vi "UHR-Fleezers Control (host) - 10.2.vi"() -> ()   [LabVIEW 2009] (continued)
            n295 = Bundle("T1 Y", "T1 X", "T1 Sum", "T2 Y", "T2 X", "T2 Sum", "T1 FB Sum", "T2 FB Sum", "PSD Y", "PSD X", "PSD Y Sum", "PSD X Sum") -> (w2177:T36)  [unwired: 1 out]
            n296 = To Word Integer(number=w2210) -> (16bit integer=w2169:i16[])
            n297 = Cluster To Array(cluster=w2177) -> (array=w2196:string[])
          }
          frame #1 {
            w2277 = 2  # Channel pattern
            # "time average x2 the 3 psd signals (detection laser)"
            # "deinterlace 3 signals from qpds"
            n298 = Decimate 1D Array(w2297) -> (w2296:i16[], w2295:i16[], w2278:i16[], w2294:i16[], w2240:i16[], w2237:i16[], w2234:i16[], w2265:i16[])
            n299 = Decimate 1D Array(w2278) -> (w2263:i16[], w2261:i16[])
            n300 = Decimate 1D Array(w2296) -> (w2293:i16[], w2280:i16[])
            n301 = Decimate 1D Array(w2295) -> (w2292:i16[], w2290:i16[])
            n302 = Decimate 1D Array(w2294) -> (w2291:i16[], w2289:i16[])
            n303 = Decimate 1D Array(w2265) -> (w2264:i16[], w2262:i16[])
            n304 = call "downsample 1D array - I16.vi"("Ave N"=2.0, "Array In"=w2240) -> ("Array Out"=w2238:i16[])  [unwired: 1 in]
            n305 = call "downsample 1D array - I16.vi"("Ave N"=2.0, "Array In"=w2234) -> ("Array Out"=w2232:i16[])  [unwired: 1 in]
            n306 = call "downsample 1D array - I16.vi"("Ave N"=2.0, "Array In"=w2237) -> ("Array Out"=w2235:i16[])  [unwired: 1 in]
            n307 = Interleave 1D Arrays(w2293, w2292, w2291, w2280, w2290, w2289, w2264, w2263, w2262, w2261, w2238, w2235, w2232) -> (w2288:i16[])
            n308 = Divide(x=w2288, y=3276.7) -> (x/y=w2287:dbl[])
            n309 = Decimate 1D Array(w2287) -> (w2286:dbl[], w2285:dbl[], w2284:dbl[], w2283:dbl[], w2282:dbl[], w2281:dbl[], w2253:dbl[], w2251:dbl[], w2250:dbl[], w2248:dbl[], w2247:dbl[], w2246:dbl[], w2243:dbl[])
            n310 = Negate(x=w2243) -> (-x=w2241:dbl[])
            n311 = Divide(x=w2247, y=w2243) -> (x/y=w2245:dbl[])
            n312 = Divide(x=w2246, y=w2241) -> (x/y=w2244:dbl[])
            n313 = Divide(x=w2286, y=w2284) -> (x/y=w2269:dbl[])
            n314 = Divide(x=w2285, y=w2284) -> (x/y=w2268:dbl[])
            n315 = Divide(x=w2283, y=w2281) -> (x/y=w2267:dbl[])
            n316 = Divide(x=w2282, y=w2281) -> (x/y=w2266:dbl[])
            n317 = Divide(x=w2253, y=w2251) -> (x/y=w2252:dbl[])
            n318 = Divide(x=w2250, y=w2248) -> (x/y=w2249:dbl[])
            n319 = Build Array(w2269, w2268, w2284, w2267, w2266, w2281, w2252, w2251, w2249, w2248, w2245, w2244, w2243) -> (w2242:dbl[][])
            n320 = Bundle("T1 Y", "T1 X", "T1 Sum", "T2 Y", "T2 X", "T2 Sum", "T1 FB X", "T1 FB Sum", "T2 FB X", "T2 FB Sum", "PSD Y", "PSD X", "PSD Y Sum") -> (w2270:T37)  [unwired: 1 out]
            n321 = Cluster To Array(cluster=w2270) -> (array=w2279:string[])
          }
          frame #2 {
            w2344 = 4  # Channel pattern
            # "time average x2 the 3 psd signals (detection laser)"
            # "deinterlace 3 signals from qpds"
            n322 = Decimate 1D Array(w2368) -> (w2367:i16[], w2366:i16[], w2345:i16[], w2365:i16[], w2311:i16[], w2357:i16[], w2356:i16[], w2333:i16[])
            n323 = Decimate 1D Array "Feedback Sum"(w2345) -> (w2329:i16[], w2327:i16[])
            n324 = Decimate 1D Array "QPD Y"(w2367) -> (w2364:i16[], w2347:i16[])
            n325 = Decimate 1D Array "QPD X"(w2366) -> (w2363:i16[], w2361:i16[])
            n326 = Decimate 1D Array "Feedback Y"(w2311) -> (w2310:i16[], w2309:i16[])
            n327 = Decimate 1D Array "QPD Sum"(w2365) -> (w2362:i16[], w2360:i16[])
            n328 = Decimate 1D Array "Feedback X"(w2333) -> (w2330:i16[], w2328:i16[])
            n329 = call "downsample 1D array - double.vi"("Ave N"=2.0, "Array In"=w2357) -> ("Array Out"=w2332:dbl[])  [unwired: 1 out]
            n330 = call "downsample 1D array - double.vi"("Ave N"=2.0, "Array In"=w2356) -> ("Array Out"=w2331:dbl[])  [unwired: 1 out]
            n331 = Interleave 1D Arrays(w2364, w2363, w2362, w2347, w2361, w2360, w2310, w2330, w2329, w2309, w2328, w2327, w2332, w2331) -> (w2355:dbl[])
            n332 = Divide(x=w2355, y=3276.7) -> (x/y=w2354:dbl[])
            n333 = Decimate 1D Array(w2354) -> (w2353:dbl[], w2352:dbl[], w2351:dbl[], w2350:dbl[], w2349:dbl[], w2348:dbl[], w2306:dbl[], w2320:dbl[], w2304:dbl[], w2305:dbl[], w2318:dbl[], w2302:dbl[], w2316:dbl[], w2314:dbl[])
            n334 = Negate(x=w2314) -> (-x=w2312:dbl[])
            n335 = Divide(x=w2316, y=w2312) -> (x/y=w2315:dbl[])
            n336 = Divide(x=w2305, y=w2302) -> (x/y=w2301:dbl[])
            n337 = Divide(x=w2306, y=w2304) -> (x/y=w2303:dbl[])
            n338 = Divide(x=w2353, y=w2351) -> (x/y=w2337:dbl[])
            n339 = Divide(x=w2352, y=w2351) -> (x/y=w2336:dbl[])
            n340 = Divide(x=w2350, y=w2348) -> (x/y=w2335:dbl[])
            n341 = Divide(x=w2349, y=w2348) -> (x/y=w2334:dbl[])
            n342 = Divide(x=w2320, y=w2304) -> (x/y=w2319:dbl[])
            n343 = Divide(x=w2318, y=w2302) -> (x/y=w2317:dbl[])
            n344 = Build Array(w2337, w2336, w2351, w2335, w2334, w2348, w2303, w2319, w2304, w2301, w2317, w2302, w2315, w2314) -> (w2313:dbl[][])
            n345 = Bundle("T1 Y", "T1 X", "T1 Sum", "T2 Y", "T2 X", "T2 Sum", "T1 FB Y", "T1 FB X", "T1 FB Sum", "T2 FB Y", "T2 FB X", "T2 FB Sum", "PSD X", "PSD Y Sum") -> (w2300:T38)  [unwired: 1 out]
            n346 = To Word Integer(number=w2355) -> (16bit integer=w2299:i16[])
            n347 = Cluster To Array(cluster=w2300) -> (array=w2346:string[])
          }
        }
      }
    }
    "AI labels" <- w866
    n348 = Decimate 1D Array(w834) -> (w862:u32[], w798:u32[])
    n349 = local read "DMA Update Period (s)"() -> (w876:dbl)
    n350 = local read "BD 1 Frequency 2 (MHz)"() -> (w737:dbl)
    n351 = local read "BD 1 Frequency 1 (MHz)"() -> (w738:dbl)
    n352 = Build Array(w862, w798) -> (w944:u32[][])
    n353 = local read "Data Period (s)"() -> (w847:dbl)
    n354 = Decimate 1D Array(w745) -> (w769:i16[], w768:i16[], w766:i16[], w765:i16[])  [unwired: 9 out]
    n355 = To Double Precision Float(number=w944) -> (double precision float=w945:dbl[][])
    n356 = local read "APD Integration Time (s)"() -> (w811:dbl)
    n357 = Divide(x=w769, y=w768) -> (x/y=w770:dbl[])
    n358 = Divide(x=w766, y=w765) -> (x/y=w767:dbl[])
    n359 = feedback #1(0.0) -> (w783:dbl)
    n360 = Add(x=w876, y=w783) -> (x+y=w984:dbl)
    n361 = local read "AOM X Cal (nm/MHz)"() -> (w735:dbl)
    n362 = To Time Stamp(1:w783) -> (0:w782:timestamp)
    n363 = Split 1D Array(array=w770, index="N El. to Ave.") -> (second subarray=w773:dbl[])  [unwired: 1 out]
    n364 = Split 1D Array(array=w767, index="N El. to Ave.") -> (second subarray=w772:dbl[])  [unwired: 1 out]
    n365 = local read "Trap X AI1 (DMA)"() -> (w771:T13)
    n366 = Multiply(x=w847, y="Trap Disp. Downsample") -> (x*y=w784:dbl)
    "Display Period (s)" <- w784
    n367 = Bundle("BD 1 Frequency 1 (MHz)"=w738, "BD 1 Frequency 2 (MHz)"=w737) -> (w739:T39)  [unwired: 1 out]
    n368 = for "Trap AI" {
      tunnel: [w2098] -> w978 mode=indexing
      tunnel: w782 -> [w2088]
      tunnel: "Trap Disp. Downsample" -> [w2096]
      tunnel: w867 -> [w2094] mode=indexing
      tunnel: w847 -> [w2093]
      tunnel: w866 -> [w2092] mode=indexing
      tunnel: w781 -> [w2091]
      tunnel: [w2090] -> w822 mode=indexing
      tunnel: w784 -> [w2089]
      workers-P: _ -> [_]
      n369 = Bundle By Name("Y"=w2094, "dt"=w2093) -> (w2095:waveform(dbl))  [unwired: 1 out]
      n370 = Set Waveform Attribute(5:w2092, 6:w2091, 7:w2095) -> (3:w2090:waveform(dbl))  [unwired: 1 in, 2 out]
      n371 = call "downsample 1D array - double.vi"("Ave N"=w2096, "Array In"=w2094) -> ("Array Out"=w2097:dbl[])  [unwired: 1 out]
      n372 = Bundle By Name(cluster=w2090, "t0"=w2088, "Y"=w2097, "dt"=w2089) -> (w2098:waveform(dbl))
    }
    n373 = call <vilib>:"Mean.vi"("X"=w772) -> ("mean"=w760:dbl)  [unwired: 1 out]
    n374 = call <vilib>:"Mean.vi"("X"=w773) -> ("mean"=w761:dbl)  [unwired: 1 out]
    n375 = Cluster To Array(cluster=w739) -> (array=w736:dbl[])
    n376 = Reciprocal(x=w784) -> (1/x=→"Trap Disp. Freq. (Hz)":dbl)
    n377 = local read "Data points/scans (MCL)"() -> (w956:dbl)
    n378 = To Fixed-Point(number=w760) -> (fixed-point=w758:fxp<+/-,16,1>)  [unwired: 1 in]
    n379 = To Fixed-Point(number=w761) -> (fixed-point=w759:fxp<+/-,16,1>)  [unwired: 1 in]
    n380 = Bundle("Trap 1 Pos.", "Trap 2 Pos.") -> (w780:cluster{string, string})  [unwired: 1 out]
    n381 = Bundle By Name(cluster=w771, "Set 1"=w759, "Set 2"=w758) -> (→"Trap X AI1 (DMA)":T13)
    n382 = Cluster To Array(cluster=w780) -> (array=w777:string[])
    n383 = for "Trap Position" {
      tunnel: w786 -> [w1028] mode=indexing
      tunnel: "Trap Disp. Downsample" -> [w1027]
      tunnel: w784 -> [w1025]
      tunnel: w782 -> [w1024]
      tunnel: w781 -> [w1022]
      tunnel: w777 -> [w1021] mode=indexing
      tunnel: [w1020] -> w734 mode=indexing
      tunnel: w736 -> [w1018] mode=indexing
      tunnel: w735 -> [w1016]
      n384 = call "downsample 1D array - double.vi"("Ave N"=w1027, "Array In"=w1028) -> ("Array Out"=w1026:dbl[])  [unwired: 1 out]
      n385 = Subtract(x=w1026, y=w1018) -> (x-y=w1019:dbl[])
      n386 = Multiply(x=w1016, y=w1019) -> (x*y=w1017:dbl[])
      n387 = Bundle By Name("Y"=w1017, "dt"=w1025, "t0"=w1024) -> (w1023:waveform(dbl))  [unwired: 1 out]
      n388 = Set Waveform Attribute(5:w1021, 6:w1022, 7:w1023) -> (3:w1020:waveform(dbl))  [unwired: 1 in, 2 out]
    }
    "Trap Positions" <- w734
    n389 = Bundle("APD 1", "APD 2") -> (w977:cluster{string, string})  [unwired: 1 out]
    n390 = Cluster To Array(cluster=w977) -> (array=w974:string[])
    n391 = for "APD" {
      tunnel: w945 -> [w2077] mode=indexing
      tunnel: w811 -> [w2085]
      tunnel: [w2081] -> w818 mode=indexing
      tunnel: "APD Disp. Scale" -> [w2082]
      tunnel: w781 -> [w2080]
      tunnel: w974 -> [w2079] mode=indexing
      tunnel: "APD Disp. Downsample" -> [w2075]
      tunnel: [w2078] -> w973
      workers-P: _ -> [_]
      tunnel: w782 -> [w2074]
      n392 = call "integrate 1D array interval - double.vi"("Ave N"=w2075, "Array In"=w2077) -> ("Array Out"=w2076:dbl[])  [unwired: 1 out]
      n393 = Multiply(x=w2085, y=w2075) -> (x*y=w2078:dbl)
      n394 = Divide(x=w2076, y=w2082) -> (x/y=w2083:dbl[])
      n395 = Bundle By Name("t0"=w2074, "Y"=w2083, "dt"=w2078) -> (w2084:waveform(dbl))  [unwired: 1 out]
      n396 = Set Waveform Attribute(5:w2079, 6:w2080, 7:w2084) -> (3:w2081:waveform(dbl))  [unwired: 1 in, 2 out]
    }
    "APD Display Period (s)" <- w973
    n397 = Reciprocal(x=w973) -> (1/x=→"APD Display Freq. (Hz)":dbl)
    n398 = local read "Display Period (s)"() -> (w846:dbl)
    n399 = Increment(x=w956) -> (x+1=w957:dbl)
    n400 = Index Array(array=w734, index=0) -> (element=w732:waveform(dbl))
    n401 = To Double Precision Float(number=w862) -> (double precision float=w861:dbl[])
    n402 = feedback #2(w957) -> (w960:dbl)
    n403 = Select(t=0, s=w947, f=w960) -> (s? t:f=w953:dbl)
    n404 = Array Size(array=w861) -> (size(s)=w959:i32)
    n405 = Add(x=w959, y=w953) -> (x+y=w954:dbl)
    n406 = Unbundle By Name(w732) -> ("Y"=w730:dbl[])
    n407 = feedback #3(w862) -> (w943:u32[])
    n408 = Build Array (concatenate)(w943, w862) -> (w940:u32[])
    n409 = feedback #4(w798) -> (w817:u32[])
    n410 = Divide(x="Bead Sep. Int. Time (s)", y=w846) -> (x/y=w728:dbl)
    n411 = Build Array (concatenate)(w817, w798) -> (w816:u32[])
    n412 = Greater?(x=w954, y=w956) -> (0:w955:bool)
    n413 = feedback #5(w730) -> (w731:dbl[])
    n414 = Build Array (concatenate)(w730, w731) -> (w729:dbl[])
    n415 = Select(t=w953, s=w955, f=w954) -> (s? t:f=w952:dbl)
    n416 = Array Size(array=w940) -> (size(s)=w937:i32)
    n417 = Array Size(array=w862) -> (size(s)=w939:i32)
    n418 = local read "MCL Scanning"() -> (w950:bool)
    n419 = local read "APD Integration Time (s)"() -> (w825:dbl)
    n420 = Build Array (concatenate)(w818, w978) -> (w820:waveform(dbl)[])
    "All Signals" <- w820
    n421 = Split 1D Array(array=w729, index=w728) -> (first subarray=w722:dbl[])  [unwired: 1 out]
    n422 = Multiply(x=w939, y="APD Ave N") -> (x*y=w938:dbl)
    n423 = Greater?(x=w937, y=w938) -> (0:w941:bool)
    n424 = Not(x=w955) -> (.not. x?=w949:bool)
    n425 = To Double Precision Float(number=w798) -> (double precision float=w797:dbl[])
    n426 = call <vilib>:"Mean.vi"("X"=w722) -> ("mean"=w721:dbl)  [unwired: 1 out]
    "Mean T1 Position (nm)" <- w721
    n427 = Subtract(x=w722, y=w721) -> (x-y=w727:dbl[])
    n428 = Square(x=w727) -> (x^2=w726:dbl[])
    n429 = And(x=w949, y=w950) -> (x .and. y?=w951:bool)
    n430 = call <vilib>:"Mean.vi"("X"=w726) -> ("mean"=w725:dbl)  [unwired: 1 out]
    n431 = case shown="True" w941 {
      tunnel: w940 -> [w1666 w1673]
      tunnel: [w1666 w1671] -> w881
      tunnel: w938 -> [_ w1668]
      tunnel: w937 -> [_ w1672]
      tunnel: w816 -> [w1665 w1670]
      tunnel: [w1665 w1667] -> w813
      frame #0 {
      }
      frame #1 {
        n432 = Subtract(x=w1672, y=w1668) -> (x-y=w1669:dbl)
        n433 = Array Subset(array=w1673, index=w1669, length=w1668) -> (w1671:u32[])
        n434 = Array Subset(array=w1670, index=w1669, length=w1668) -> (w1667:u32[])
      }
    }
    n435 = Or(x=w951, y=w947) -> (x .or. y?=w948:bool)
    n436 = Square Root(x=w725) -> (sqrt(x)=w724:dbl)
    n437 = Equal?(x="Tab Control 6", y=T26."High Res Display") -> (x = y?=w870:bool)
    n438 = Multiply(x="APD Disp. Scale", y=w818) -> (x*y=w827:waveform(dbl)[])
    n439 = Multiply(x="APD Disp. Downsample", y=w825) -> (x*y=w823:dbl)
    n440 = Multiply(x=10.0, y=w724) -> (x*y=→"Trap 1 Position RMS (A)":dbl)
    n441 = Divide(x=w827, y=w823) -> (x/y=w795:waveform(dbl)[])
    n442 = Index Array(array=w795, index=0) -> (element=w805:waveform(dbl))
    n443 = case "For computing FFTs for display" shown="True" "Compute FFT" {
      tunnel: w822 -> [_ w2873]
      frame #0 {
      }
      frame #1 {
        n444 = Build Array("FFT 1 Choice 1", "FFT 1 Choice 2", "FFT 2 Choice 1", "FFT 2 Choice 2") -> (w2866:u16[])
        n445 = Array Size(array=w2873) -> (size(s)=w2872:i32)
        n446 = feedback #6(u16[] [100, 100, 100, 100]) -> (w2867:u16[])
        n447 = feedback #7("# Spectra to Ave.") -> (w2864:dbl)
        n448 = Not Equal?(x="# Spectra to Ave.", y=w2864) -> (x != y?=w2863:bool)
        n449 = Not Equal?(x=w2866, y=w2867) -> (x != y?=w2865:bool)
        n450 = feedback #8(1.0) -> (w2850:dbl)
        n451 = Compound Arithmetic op=OR("Reset FFT", w2865, w2863) -> (w2848:bool)
        n452 = Select(t=1.0, s=w2848, f=w2850) -> (s? t:f=w2852:dbl)
        n453 = Greater?(x=w2852, y="# Spectra to Ave.") -> (0:w2871:bool)
        n454 = Increment(x=w2852) -> (x+1=w2851:dbl)
        n455 = local read "DMA Update Period (s)"() -> (w2846:dbl)
        n456 = Multiply(x="# Spectra to Ave.", y=w2846) -> (x*y=→"Ave. Time (s)":dbl)
        n457 = Build Array(cluster{"f0":dbl, "df":dbl, "magnitude":dbl[]} {"f0"=0.0, "df"=0.0, "magnitude"=[]} ("PSD")) -> (w2855:cluster{"f0":dbl, "df":dbl, "magnitude":dbl[]}[])
        n458 = Build Array(w2855, w2855, w2855, w2855) -> (w2857:T40)
        n459 = feedback #9(w2857) -> (w2862:T40)
        n460 = for {
          N: 4 -> [_]
          tunnel: w2866 -> [w2895] mode=indexing
          tunnel: w2873 -> [w2896]
          tunnel: w2872 -> [w2898]
          tunnel: w2848 -> [w2891]
          tunnel: w2871 -> [w2890]
          tunnel: "# Spectra to Ave." -> [w2889]
          tunnel: [w2888] -> w2861 mode=indexing
          tunnel: w2862 -> [w2893] mode=indexing
          tunnel: [w2892] -> w2849 mode=indexing
          tunnel: w2852 -> [w2887]
          n461 = Less?(x=w2895, y=w2898) -> (x < y?=w2897:bool)
          n462 = Index Array(array=w2896, index=w2895) -> (element=w2894:waveform(dbl))
          n463 = case shown="True" w2897 {
            tunnel: w2894 -> [_ w2915]
            tunnel: w2893 -> [w2900 w2913]
            tunnel: [w2900 w2901] -> w2892
            tunnel: w2891 -> [_ w2912]
            tunnel: w2890 -> [_ w2905]
            tunnel: w2889 -> [_ w2904]
            tunnel: [cluster{"f0":dbl, "df":dbl, "magnitude":dbl[]} {"f0"=0.0, "df"=0.0, "magnitude"=[]} ("PSD") w2906] -> w2888
            tunnel: w2887 -> [_ w2903]
            frame #0 {
            }
            frame #1 {
              n464 = call <vilib>:"Std Deviation and Variance.vi"("X"=w2915) -> ("mean"=w2916:dbl)  [unwired: 1 in, 2 out]
              n465 = Subtract(x=w2915, y=w2916) -> (x-y=w2914:waveform(dbl))
              n466 = xnode "Spectral Measurements"("Signals"=w2914) -> ("PSD"=w2908:cluster{"f0":dbl, "df":dbl, "magnitude":dbl[]})  [unwired: 1 in, 1 out]
              n467 = case shown="False" w2912 {
                tunnel: w2913 -> [w2925 _]
                tunnel: [w2921 w2930] -> w2901
                tunnel: w2908 -> [w2924 w2931]
                tunnel: w2905 -> [w2923 _]
                frame #0 {
                  n468 = Build Array (concatenate)(w2925, w2924) -> (w2922:cluster{"f0":dbl, "df":dbl, "magnitude":dbl[]}[])
                  n469 = case shown="True" w2923 {
                    tunnel: w2922 -> [w2926 w2929]
                    tunnel: [w2926 w2927] -> w2921
                    frame #0 {
                    }
                    frame #1 {
                      n470 = Delete From Array(array=w2929, index=0) -> (array with subset deleted=w2927:cluster{"f0":dbl, "df":dbl, "magnitude":dbl[]}[])  [unwired: 1 in, 1 out]
                    }
                  }
                }
                frame #1 {
                  n471 = Build Array(w2931) -> (w2930:cluster{"f0":dbl, "df":dbl, "magnitude":dbl[]}[])
                }
              }
              n472 = for {
                tunnel: w2901 -> [w2920] mode=indexing
                tunnel: [w2919] -> w2911 mode=indexing
                workers-P: _ -> [_]
                n473 = Unbundle By Name(w2920) -> ("magnitude"=w2919:dbl[])
              }
              n474 = Transpose 2D Array(2D array=w2911) -> (transposed array=w2910:dbl[][])
              n475 = for {
                tunnel: w2910 -> [w2918] mode=indexing
                tunnel: [w2917] -> w2909 mode=indexing
                workers-P: _ -> [_]
                n476 = Add Array Elements(numeric array=w2918) -> (sum=w2917:dbl)
              }
              n477 = Select(t=w2904, s=w2905, f=w2903) -> (s? t:f=w2902:dbl)
              n478 = Divide(x=w2909, y=w2902) -> (x/y=w2907:dbl[])
              n479 = Bundle By Name(cluster=w2908, "magnitude"=w2907) -> (w2906:cluster{"f0":dbl, "df":dbl, "magnitude":dbl[]})
            }
          }
        }
        n480 = case shown="True" w2848 {
          tunnel: w2849 -> [w2880 w2886]
          tunnel: [w2880 w2881] -> w2847
          frame #0 {
          }
          frame #1 {
            n481 = Array Subset(array=w2886, index (row)=0 ("index"), length (row)=4 ("length"), index (col)=0 ("index"), length (col)=1 ("length")) -> (w2881:T40)
          }
        }
        n482 = Split 1D Array(array=w2861, index=2) -> (first subarray=→"FFT 1":cluster{"f0":dbl, "df":dbl, "magnitude":dbl[]}[], second subarray=→"FFT 2":cluster{"f0":dbl, "df":dbl, "magnitude":dbl[]}[])
      }
    }
    n483 = Index Array(array=w795, index=1) -> (element=w803:waveform(dbl))
    n484 = case "For displaying the high resolution display (no downsampling)" shown="True" w870 {
      tunnel: w822 -> [_ w1192]
      frame #0 {
      }
      frame #1 {
        n485 = Index Array(array=w1192, index="High Res. Display") -> (element=w1193:waveform(dbl))
        n486 = call <vilib>:"Std Deviation and Variance.vi"("X"=w1193) -> ("mean"=w1200:dbl, "standard deviation"=w1205:dbl)  [unwired: 1 in, 1 out]
        "Mean Intensity" <- w1200
        "Sigma" <- w1205
        n487 = Subtract(x=w1193, y=w1200) -> (x-y=w1199:waveform(dbl))
        n488 = Select(t=w1199, s="Subtract mean", f=w1193) -> (s? t:f=→"1 Channel":waveform(dbl))
        n489 = Divide(x=w1205, y=w1200) -> (x/y=→"Sigma/Mean":dbl)
        n490 = feedback #10(1) -> (w1194:i32)
        n491 = Greater Or Equal?(x=w1194, y="Slow mean N ave.") -> (x >= y?=w1207:bool)
        n492 = Increment(x=w1194) -> (x+1=w1209:i32)
        n493 = Select(t=1, s=w1207, f=w1209) -> (s? t:f=w1196:i32)
        n494 = feedback #11() -> (w1197:waveform(dbl))  [unwired: 1 out]
        n495 = case shown="Default" w1194 {
          tunnel: [w1212 w1215] -> w1198
          tunnel: w1197 -> [w1214 _]
          tunnel: w1193 -> [w1213 w1215]
          frame #0 {
            n496 = call-poly <vilib>:"Append Waveforms.vi"("waveform B"=w1213, "waveform A"=w1214) -> ("waveform out"=w1212:waveform(dbl))  [unwired: 1 in, 8 out]
          }
          frame #1 {
          }
        }
        n497 = case shown="True" w1207 {
          tunnel: w1198 -> [_ w1211]
          frame #0 {
          }
          frame #1 {
            n498 = call <vilib>:"Mean.vi"("X"=w1211) -> ("mean"=→"Slow mean":dbl)  [unwired: 1 out]
          }
        }
      }
    }
    n499 = case "For plotting results of scanning MCL" shown="True" w948 {
      tunnel: w947 -> [_ w1706]
      tunnel: w861 -> [_ w1802]
      tunnel: w956 -> [_ _]
      tunnel: w822 -> [_ w1776]
      tunnel: w797 -> [_ w1707]
      tunnel: w796 -> [_ w1680]
      frame #0 {
      }
      frame #1 {
        w1687 = u32 0 items=["Horizontal", "Vertical", "Central", "1st Diagonal", "2nd Diagonal"] ("Type of Symmetry")
        w1715 = u32 0 items=["Horizontal", "Vertical", "Central", "1st Diagonal", "2nd Diagonal"] ("Type of Symmetry")
        w1718 = u32 0 items=["Horizontal", "Vertical", "Central", "1st Diagonal", "2nd Diagonal"] ("Type of Symmetry")
        w1747 = u32 0 items=["Horizontal", "Vertical", "Central", "1st Diagonal", "2nd Diagonal"] ("Type of Symmetry")
        n500 = Index Array(array=w1776, index=10) -> (element=w1782:waveform(dbl))
        n501 = Index Array(array=w1776, index=11) -> (element=w1779:waveform(dbl))
        n502 = Index Array(array=w1776, index="Channel") -> (element=w1778:waveform(dbl))
        n503 = local read "Cycles/step (MCL)"() -> (w1732:u64)
        n504 = Unbundle(w1680) -> ("New Image"=w1679:T2, "New Image"=w1678:T2, "New Image"=w1677:T2, "New Image"=w1676:T2)
        n505 = Unbundle By Name(w1782) -> ("Y"=w1734:dbl[])
        n506 = Unbundle By Name(w1779) -> ("Y"=w1736:dbl[])
        n507 = Unbundle By Name(w1778) -> ("Y"=w1741:dbl[])
        n508 = call "downsample 1D array - double.vi"("Ave N"=w1732, "Array In"=w1734) -> ("Array Out"=w1733:dbl[])  [unwired: 1 out]
        n509 = call "downsample 1D array - double.vi"("Ave N"=w1732, "Array In"=w1736) -> ("Array Out"=w1735:dbl[])  [unwired: 1 out]
        n510 = call "downsample 1D array - double.vi"("Ave N"=w1732, "Array In"=w1741) -> ("Array Out"=w1740:dbl[])  [unwired: 1 out]
        n511 = feedback #12(w1802) -> (w1803:dbl[])
        n512 = Build Array (concatenate)(w1803, w1802) -> (w1784:dbl[])
        n513 = feedback #13(w1707) -> (w1709:dbl[])
        n514 = Build Array (concatenate)(w1709, w1707) -> (w1708:dbl[])
        n515 = Select(t=w1802, s=w1706, f=w1784) -> (s? t:f=w1788:dbl[])
        n516 = local read "Scan steps (MCL)"() -> (w1689:u64)
        n517 = Select(t=w1707, s=w1706, f=w1708) -> (s? t:f=w1690:dbl[])
        n518 = local read "Scan lines (y)"() -> (w1675:u64)
        n519 = local read "N APD Samp/step"() -> (w1691:dbl)
        n520 = feedback #14(w1733) -> (w1790:dbl[])
        n521 = Build Array (concatenate)(w1790, w1733) -> (w1781:dbl[])
        n522 = feedback #15(w1740) -> (w1800:dbl[])
        n523 = Build Array (concatenate)(w1800, w1740) -> (w1799:dbl[])
        n524 = feedback #16(w1735) -> (w1792:dbl[])
        n525 = Build Array (concatenate)(w1792, w1735) -> (w1793:dbl[])
        n526 = Select(t=w1733, s=w1706, f=w1781) -> (s? t:f=w1737:dbl[])
        n527 = Select(t=w1740, s=w1706, f=w1799) -> (s? t:f=w1739:dbl[])
        n528 = Select(t=w1735, s=w1706, f=w1793) -> (s? t:f=w1738:dbl[])
        n529 = Multiply(x=w1689, y=u64 2) -> (x*y=w1674:u64)
        n530 = call "integrate 1D array interval - double.vi"("Ave N"=w1691, "Array In"=w1690) -> ("Array Out"=w1702:dbl[])  [unwired: 1 out]
        n531 = call "integrate 1D array interval - double.vi"("Ave N"=w1691, "Array In"=w1788) -> ("Array Out"=w1787:dbl[])  [unwired: 1 out]
        n532 = Array Size(array=w1702) -> (size(s)=w1703:i32)
        n533 = Array Size(array=w1787) -> (size(s)=w1789:i32)
        n534 = Multiply(x=w1675, y=w1674) -> (x*y=w1705:u64)
        n535 = Multiply(x=w1675, y=w1674) -> (x*y=w1797:u64)
        n536 = call <vilib>:"Mean.vi"("X"=w1737) -> ("mean"=w1721:dbl)  [unwired: 1 out]
        n537 = Subtract(x=w1705, y=w1703) -> (x-y=w1696:u64)
        n538 = call <vilib>:"Mean.vi"("X"=w1739) -> ("mean"=w1726:dbl)  [unwired: 1 out]
        n539 = call <vilib>:"Mean.vi"("X"=w1738) -> ("mean"=w1724:dbl)  [unwired: 1 out]
        n540 = call <vilib>:"Mean.vi"("X"=w1702) -> ("mean"=w1693:dbl)  [unwired: 1 out]
        n541 = Subtract(x=w1797, y=w1789) -> (x-y=w1731:u64)
        n542 = call <vilib>:"Mean.vi"("X"=w1787) -> ("mean"=w1728:dbl)  [unwired: 1 out]
        n543 = Initialize Array(1.0 ("element"), w1696) -> (w1692:dbl[])
        n544 = Initialize Array(1.0 ("element"), w1731) -> (w1722:dbl[])
        n545 = Multiply(x=w1692, y=w1693) -> (x*y=w1694:dbl[])
        n546 = Multiply(x=w1722, y=w1724) -> (x*y=w1725:dbl[])
        n547 = Multiply(x=w1722, y=w1726) -> (x*y=w1727:dbl[])
        n548 = Multiply(x=w1722, y=w1721) -> (x*y=w1723:dbl[])
        n549 = Multiply(x=w1722, y=w1728) -> (x*y=w1729:dbl[])
        n550 = Build Array (concatenate)(w1737, w1723) -> (w1791:dbl[])
        n551 = Build Array (concatenate)(w1739, w1727) -> (w1795:dbl[])
        n552 = Build Array (concatenate)(w1738, w1725) -> (w1794:dbl[])
        n553 = Build Array (concatenate)(w1702, w1694) -> (w1704:dbl[])
        n554 = Build Array (concatenate)(w1787, w1729) -> (w1796:dbl[])
        n555 = Reshape Array(w1791, w1675, w1674) -> (w1757:dbl[][])
        n556 = Reshape Array(w1704, w1675, w1674) -> (w1700:dbl[][])
        n557 = Reshape Array(w1795, w1675, w1674) -> (w1749:dbl[][])
        n558 = Reshape Array(w1794, w1675, w1674) -> (w1764:dbl[][])
        n559 = Reshape Array(w1796, w1675, w1674) -> (w1774:dbl[][])
        n560 = Array Subset(array=w1764, index (col)=0 ("index"), length (col)=w1689) -> (w1769:dbl[][])  [unwired: 2 in]
        n561 = Array Subset(array=w1764, index (col)=w1689) -> (w1767:dbl[][])  [unwired: 3 in]
        n562 = Array Subset(array=w1749, index (col)=0 ("index"), length (col)=w1689) -> (w1755:dbl[][])  [unwired: 2 in]
        n563 = Array Subset(array=w1749, index (col)=w1689) -> (w1753:dbl[][])  [unwired: 3 in]
        n564 = Array Subset(array=w1700, index (col)=0 ("index"), length (col)=w1689) -> (w1699:dbl[][])  [unwired: 2 in]
        n565 = Array Subset(array=w1700, index (col)=w1689) -> (w1697:dbl[][])  [unwired: 3 in]
        n566 = Array Subset(array=w1774, index (col)=0 ("index"), length (col)=w1689) -> (w1773:dbl[][])  [unwired: 2 in]
        n567 = Array Subset(array=w1774, index (col)=w1689) -> (w1771:dbl[][])  [unwired: 3 in]
        n568 = Array Subset(array=w1757, index (col)=0 ("index"), length (col)=w1689) -> (w1762:dbl[][])  [unwired: 2 in]
        n569 = Array Subset(array=w1757, index (col)=w1689) -> (w1760:dbl[][])  [unwired: 3 in]
        n570 = for {
          tunnel: w1769 -> [w1811] mode=indexing
          tunnel: [w1810] -> w1768 mode=indexing
          workers-P: _ -> [_]
          n571 = Reverse 1D Array(array=w1811) -> (reversed array=w1810:dbl[])
        }
        n572 = for {
          tunnel: w1755 -> [w1807] mode=indexing
          tunnel: [w1806] -> w1754 mode=indexing
          workers-P: _ -> [_]
          n573 = Reverse 1D Array(array=w1807) -> (reversed array=w1806:dbl[])
        }
        n574 = for {
          tunnel: w1699 -> [w1805] mode=indexing
          tunnel: [w1804] -> w1698 mode=indexing
          workers-P: _ -> [_]
          n575 = Reverse 1D Array(array=w1805) -> (reversed array=w1804:dbl[])
        }
        n576 = for {
          tunnel: w1773 -> [w1813] mode=indexing
          tunnel: [w1812] -> w1772 mode=indexing
          workers-P: _ -> [_]
          n577 = Reverse 1D Array(array=w1813) -> (reversed array=w1812:dbl[])
        }
        n578 = for {
          tunnel: w1762 -> [w1809] mode=indexing
          tunnel: [w1808] -> w1761 mode=indexing
          workers-P: _ -> [_]
          n579 = Reverse 1D Array(array=w1809) -> (reversed array=w1808:dbl[])
        }
        n580 = Index Array(array=w1774, index (row)=0) -> (element=→"Waveform Graph":dbl[])  [unwired: 1 in]
        n581 = Add(x=w1768, y=w1767) -> (x+y=w1766:dbl[][])
        n582 = Add(x=w1754, y=w1753) -> (x+y=w1752:dbl[][])
        n583 = Add(x=w1698, y=w1697) -> (x+y=w1682:dbl[][])
        n584 = Add(x=w1772, y=w1771) -> (x+y=w1746:dbl[][])
        n585 = Add(x=w1761, y=w1760) -> (x+y=w1759:dbl[][])
        n586 = Divide(x=w1752, y=2) -> (x/y=w1750:dbl[][])
        n587 = Divide(x=w1766, y=2) -> (x/y=w1711:dbl[][])
        n588 = Divide(x=w1759, y=2) -> (x/y=w1713:dbl[][])
        n589 = To Single Precision Float(number=w1746) -> (single precision float=w1745:sgl[][])
        n590 = Transpose 2D Array(2D array=w1750) -> (transposed array=→"Data map":dbl[][])
        n591 = To Single Precision Float(number=w1682) -> (single precision float=w1686:sgl[][])
        n592 = To Single Precision Float(number=w1711) -> (single precision float=w1717:sgl[][])
        n593 = To Single Precision Float(number=w1713) -> (single precision float=w1714:sgl[][])
        n594 = call "IMAQ ArrayToImage"("Image Pixels (Float)"=w1745, "Image"=w1679) -> ("Image Out"=w1748:T2)  [unwired: 8 in, 1 out]
        n595 = call "IMAQ ArrayToImage"("Image Pixels (Float)"=w1686, "Image"=w1678) -> ("Image Out"=w1688:T2)  [unwired: 8 in, 1 out]
        n596 = call "IMAQ ArrayToImage"("Image Pixels (Float)"=w1717, "Image"=w1677) -> ("Image Out"=w1719:T2)  [unwired: 8 in, 1 out]
        n597 = call "IMAQ ArrayToImage"("Image Pixels (Float)"=w1714, "Image"=w1676) -> ("Image Out"=w1716:T2)  [unwired: 8 in, 1 out]
        n598 = call "IMAQ Symmetry"("Type of Symmetry"=w1747, "Image Src"=w1748) -> ("Image Dst Out"=w1743:T2)  [unwired: 3 in, 1 out]
        n599 = call "IMAQ Symmetry"("Type of Symmetry"=w1687, "Image Src"=w1688) -> ("Image Dst Out"=w1684:T2)  [unwired: 3 in, 1 out]
        n600 = call "IMAQ Symmetry"("Type of Symmetry"=w1718, "Image Src"=w1719) -> ("Image Dst Out"=→"Detection Laser X":T2)  [unwired: 3 in, 1 out]
        n601 = call "IMAQ Symmetry"("Type of Symmetry"=w1715, "Image Src"=w1716) -> ("Image Dst Out"=→"Detection Laser Y":T2)  [unwired: 3 in, 1 out]
        n602 = call "IMAQ Set Simple Calibration"("Calibration Axis Info"=T27 {"Origin Pixel"={"X"=0.0, "Y"=0.0}, "Angle Relative to Horizontal (deg)"=0.0, "Axis Reference"=0}, "Grid Descriptor"=T28 {"X Step"=0.3, "Y Step"=0.3, "Unit"=enum."Undefined"}, "Image"=w1743) -> ("Calibrated Image"=→"APD 1":T2)  [unwired: 7 in, 1 out]
        n603 = call "IMAQ Set Simple Calibration"("Calibration Axis Info"=T27 {"Origin Pixel"={"X"=0.0, "Y"=0.0}, "Angle Relative to Horizontal (deg)"=0.0, "Axis Reference"=0}, "Grid Descriptor"=T28 {"X Step"=0.3, "Y Step"=0.3, "Unit"=enum."Undefined"}, "Image"=w1684) -> ("Calibrated Image"=→"APD 2":T2)  [unwired: 7 in, 1 out]
      }
    }
    n604 = Subtract(x=w803, y="APD 2 Offset") -> (x-y=w800:waveform(dbl))
    n605 = Subtract(x=w805, y="APD 1 Offset") -> (x-y=w801:waveform(dbl))
    n606 = Index Array(array=w820, index=3) -> (element=w892:waveform(dbl))
    n607 = Index Array(array=w820, index=6) -> (element=w889:waveform(dbl))
    n608 = Build Array(w801, w800) -> (→"APD Chart":waveform(dbl)[])
    n609 = Array Size(array=w881) -> (size(s)=w936:i32)
    n610 = call <vilib>:"Std Deviation and Variance.vi"("X"=w813) -> ("standard deviation"=w812:dbl)  [unwired: 1 in, 2 out]
    n611 = Add Array Elements(numeric array=w813) -> (sum=w815:u32)
    n612 = Add Array Elements(numeric array=w881) -> (sum=w946:u32)
    n613 = call <vilib>:"Std Deviation and Variance.vi"("X"=w881) -> ("standard deviation"=w880:dbl)  [unwired: 1 in, 2 out]
    n614 = Divide(x="T1 offset_x (mV)", y=1000.0) -> (x/y=w893:dbl)
    n615 = Divide(x=w812, y=w811) -> (x/y=w808:dbl)
    "Rate sigma (Hz) 2" <- w808
    n616 = Multiply(x=w811, y=w936) -> (x*y=w814:dbl)
    "Int. Time (s)" <- w814
    n617 = Divide(x=w815, y=w814) -> (x/y=w809:dbl)
    "APD 2 Rate (Hz)" <- w809
    n618 = Divide(x=w946, y=w814) -> (x/y=w878:dbl)
    "APD 1 Rate (Hz)" <- w878
    n619 = Divide(x=w880, y=w811) -> (x/y=w879:dbl)
    "Rate sigma (Hz)" <- w879
    n620 = Divide(x=w808, y=w809) -> (x/y=→"Sigma/Mean 2":dbl)
    n621 = Divide(x=w879, y=w878) -> (x/y=→"Sigma/Mean":dbl)
    n622 = Divide(x="T2 offset_x (mV)", y=1000.0) -> (x/y=w891:dbl)
    n623 = case shown="0, Default" "Calibration" {
      tunnel: "T1 alpha_x (nm/V)" -> [_ w1642 w1663]
      tunnel: "T1 kappa_x (pN/nm)" -> [_ _ w1653]
      tunnel: "T2 alpha_x (nm/V)" -> [_ w1641 w1661]
      tunnel: "T2 kappa_x (pN/nm)" -> [_ _ w1654]
      tunnel: w892 -> [w1624 w1639 w1659]
      tunnel: w889 -> [w1623 w1637 w1657]
      tunnel: [w1624 w1636 w1656] -> w922
      tunnel: [w1623 w1635 w1655] -> w921
      tunnel: ["T1 X (V)" ("Label.Text") "T1 X (nm)" ("Label.Text") "T1 X (pN)" ("Label.Text")] -> w910
      tunnel: ["T2 X (V)" ("Label.Text") "T2 X (nm)" ("Label.Text") "T2 X (pN)" ("Label.Text")] -> w909
      tunnel: ["Position (V)" ("Label.Text") "Position (nm)" ("Label.Text") "Force (pN)" ("Label.Text")] -> w911
      tunnel: w891 -> [_ w1627 w1646]
      tunnel: w893 -> [_ w1630 w1648]
      tunnel: ["Mean (V)" ("Label.Text") "Mean (nm)" ("Label.Text") "Mean (pN)" ("Label.Text")] -> w906
      tunnel: ["Difference (V)" ("Label.Text") "Difference (nm)" ("Label.Text") "Difference (pN)" ("Label.Text")] -> w828
      frame #0 {
      }
      frame #1 {
        n624 = Unbundle By Name(w1639) -> ("Y"=w1643:dbl[])
        n625 = Unbundle By Name(w1637) -> ("Y"=w1628:dbl[])
        n626 = Subtract(x=w1643, y=w1630) -> (x-y=w1631:dbl[])
        n627 = Subtract(x=w1628, y=w1627) -> (x-y=w1629:dbl[])
        n628 = Multiply(x=w1629, y=w1641) -> (x*y=w1638:dbl[])
        n629 = Multiply(x=w1642, y=w1631) -> (x*y=w1640:dbl[])
        n630 = Bundle By Name(cluster=w1637, "Y"=w1638) -> (w1635:waveform(dbl))
        n631 = Bundle By Name(cluster=w1639, "Y"=w1640) -> (w1636:waveform(dbl))
      }
      frame #2 {
        n632 = Unbundle By Name(w1659) -> ("Y"=w1664:dbl[])
        n633 = Unbundle By Name(w1657) -> ("Y"=w1662:dbl[])
        n634 = Subtract(x=w1662, y=w1646) -> (x-y=w1647:dbl[])
        n635 = Subtract(x=w1664, y=w1648) -> (x-y=w1649:dbl[])
        n636 = Compound Arithmetic op=MULTIPLY(w1647, w1661, w1654) -> (w1658:dbl[])
        n637 = Compound Arithmetic op=MULTIPLY(w1653, w1663, w1649) -> (w1660:dbl[])
        n638 = Bundle By Name(cluster=w1657, "Y"=w1658) -> (w1655:waveform(dbl))
        n639 = Bundle By Name(cluster=w1659, "Y"=w1660) -> (w1656:waveform(dbl))
      }
    }
    n640 = feedback #17(u16 1 ("Calibration")) -> (w913:u16)
    n641 = Not Equal?(x=w913, y="Calibration") -> (x != y?=w868:bool)
    n642 = Unbundle By Name(w892) -> ("Y"=w895:dbl[])
    n643 = Unbundle By Name(w889) -> ("Y"=w898:dbl[])
    n644 = Subtract(x=w895, y=w893) -> (x-y=w896:dbl[])
    n645 = Subtract(x=w898, y=w891) -> (x-y=w897:dbl[])
    n646 = Multiply(x=w897, y="T2 alpha_x (nm/V)") -> (x*y=w888:dbl[])
    n647 = Multiply(x="T1 alpha_x (nm/V)", y=w896) -> (x*y=w887:dbl[])
    n648 = Multiply(x=w921, y=-1.0) -> (x*y=w900:waveform(dbl))
    n649 = case shown="True" "Read Lateness and Rel Phase" {
      tunnel: w864 -> [w1216 w1238]
      tunnel: w863 -> [w1217 w1237]
      tunnel: [w1216 w1236] -> w884
      tunnel: [w1217 w1235] -> w883
      frame #0 {
      }
      frame #1 {
        n650 = xnode "Read/Write Control"("FPGA VI Reference In"=w1238, "error in"=w1237) -> ("FPGA VI Reference Out"=w1236:T21, "error out"=w1235:errorcluster, "GI Relative phase"=→"GI relative phase":i16, "Relative phase"=→"Relative phase (AI1)":i16, "AI Late Counter"=→"Late Counter (AI1)":u16, "GI Late Counter"=→"GI Late Counter":u16, "MCL Late Counter"=→"MCL Late Counter":u16, "MCL Relative Phase"=→"Relative Phase (MCL)":i16, "APD Acq Relative Phase"=→"APD Acq Relative Phase":i16, "APD 1 Gate Relative Phase"=→"APD 1 Gate Relative Phase":i16, "APD 2 Gate Relative Phase"=→"APD 2 Gate Relative Phase":i16, "APD Acq Late Counter"=→"APD Acq Late Counter":u16, "APD 1 Gate Late Counter"=→"APD 1 Gate Late Counter":u16, "APD 2 Gate Late Counter"=→"APD 2 Gate Late Counter":u16, "Green FB Relative Phase"=→"Relative phase (Green FB)":i16, "GI Relative phase 2"=→"GI relative phase 2":i16, "GI Late Counter 2"=→"GI Late Counter 2":u16, "Trap Pos FIFO Timeout"=→"Trap Pos FIFO Timeout":u16, "Trap AI FIFO Timeout"=→"Trap AI FIFO Timeout":u16)
      }
    }
    n651 = Subtract(x=w888, y=w887) -> (x-y=w886:dbl[])
    n652 = Unbundle By Name(w921) -> ("Y"=w853:dbl[])
    n653 = Unbundle By Name(w922) -> ("Y"=w854:dbl[])
    n654 = Build Array(w922, w900) -> (→"Force":waveform(dbl)[])
    n655 = Subtract(x=w886, y="Offset (nm)") -> (x-y=w851:dbl[])
    n656 = call <vilib>:"Mean.vi"("X"=w853) -> ("mean"=w832:dbl)  [unwired: 1 out]
    "T2 X" <- w832
    n657 = Absolute Value(x=w854) -> (abs(x)=w855:dbl[])
    n658 = Absolute Value(x=w853) -> (abs(x)=w856:dbl[])
    n659 = call <vilib>:"Mean.vi"("X"=w854) -> ("mean"=w833:dbl)  [unwired: 1 out]
    "T1 X" <- w833
    n660 = Add(x=w855, y=w856) -> (x+y=w857:dbl[])
    n661 = Bundle By Name(cluster=w892, "Y"=w851) -> (w819:waveform(dbl))
    "Bead Separation" <- w819
    n662 = Divide(x=w857, y=2.0) -> (x/y=→"Vec Mean of T1 T2":dbl[])
    n663 = case shown="True" w868 {
      tunnel: w911 -> [_ w1617]
      tunnel: w910 -> [_ w1616]
      tunnel: w909 -> [_ w1615]
      tunnel: w906 -> [_ w1614]
      tunnel: w828 -> [_ w1613]
      frame #0 {
      }
      frame #1 {
        n664 = property on="Force" class="WFChart (strict)"("YScale.NameLbl.Text"=w1617) -> ()  [unwired: 2 in, 2 out]
        n665 = property on="T2 X" class="DigNum (strict)"("Caption.Text"=w1615) -> ()  [unwired: 2 in, 2 out]
        n666 = property on="T1 X" class="DigNum (strict)"("Caption.Text"=w1616) -> ()  [unwired: 2 in, 2 out]
        n667 = property on="Mean" class="DigNum (strict)"("Caption.Text"=w1614) -> ()  [unwired: 2 in, 2 out]
        n668 = property on="Difference" class="DigNum (strict)"("Caption.Text"=w1613) -> ()  [unwired: 2 in, 2 out]
      }
    }
    n669 = local read "Tether"() -> (w860:bool)
    n670 = Absolute Value(x=w833) -> (abs(x)=w830:dbl)
    n671 = Absolute Value(x=w832) -> (abs(x)=w829:dbl)
    n672 = Add(x=w830, y=w829) -> (x+y=w908:dbl)
    n673 = Subtract(x=w830, y=w829) -> (x-y=→"Difference":dbl)
    n674 = feedback #18(w851) -> (w850:dbl[])
    n675 = Divide(x=w908, y=2.0) -> (x/y=w859:dbl)
    "Mean" <- w859
    n676 = case shown="True" w860 {
      tunnel: w859 -> [_ w1175]
      frame #0 {
      }
      frame #1 {
        n677 = Greater?(x="Lost Tether Alarm Threshold (pN)", y=w1175) -> (0:w1173:bool)
        n678 = case shown="True" w1173 {
          frame #0 {
          }
          frame #1 {
            n679 = flat-sequence {
              frame #0 {
                # "stop only if saving"
                n680 = local read "Saving..."() -> (w1188:bool)
                n681 = And(x=w1188, y="TA Cancel Save?") -> (x .and. y?=w1187:bool)
                n682 = local write "Stop Saving"(w1187) -> ()
              }
              frame #1 {
                n683 = case shown="True" "TA Green Off?" {
                  frame #0 {
                  }
                  frame #1 {
                    w1191 = FALSE ("Fl. Triggered...")
                    n684 = local write "Fl. Triggered..."(w1191) -> ()
                    n685 = property on="Green Laser ON/Interlacing" class="Bool (strict)"("Val(Sgnl)"=w1191) -> ()  [unwired: 2 in, 2 out]
                  }
                }
              }
            }
            n686 = local read "Time tether formed"() -> (w1182:timestamp)
            n687 = Get Date/Time In Seconds() -> (seconds since 1Jan1904=w1183:timestamp)
            n688 = Subtract(x=w1183, y=w1182) -> (x-y=w1181:dbl)
            n689 = Number To Decimal String(number=w1181) -> (decimal integer string=w1178:string)  [unwired: 1 out]
            n690 = local read "Messages"() -> (w1185:string)
            n691 = call <vilib>:"Beep.vi"() -> ()  [unwired: 3 in, 9 out]
            n692 = Concatenate Strings("Lost tether (" ("Message to add"), w1178, " s)." ("string")) -> (w1180:string)
            n693 = local write "Tether"(FALSE ("Tether")) -> ()
            n694 = call "Update messages.vi"("Message to add"=w1180, "Old message string"=w1185) -> ("New message string"=w1184:string)
            n695 = local write "Messages"(w1184) -> ()
            n696 = property on="Trap Pos. FB ON" class="Bool (strict)"("Val(Sgnl)"=FALSE ("Value (Signaling)")) -> ()  [unwired: 2 in, 2 out]
          }
        }
      }
    }
    n697 = Build Array (concatenate)(w851, w850) -> (w849:dbl[])
    n698 = Split 1D Array(array=w849, index=w728) -> (first subarray=w845:dbl[])  [unwired: 1 out]
    n699 = call <vilib>:"Mean.vi"("X"=w845) -> ("mean"=w844:dbl)  [unwired: 1 out]
    "Bead Mean (nm)" <- w844
    n700 = Subtract(x=w845, y=w844) -> (x-y=w843:dbl[])
    n701 = Square(x=w843) -> (x^2=w842:dbl[])
    n702 = call <vilib>:"Mean.vi"("X"=w842) -> ("mean"=w841:dbl)  [unwired: 1 out]
    n703 = Square Root(x=w841) -> (sqrt(x)=w840:dbl)
    n704 = Multiply(x=10.0, y=w840) -> (x*y=→"RMS (Ang)":dbl)
    n705 = xnode "Read/Write Control"("FPGA VI Reference In"=w884, "error in"=w883) -> ("FPGA VI Reference Out"=w1002:T21, "error out"=w996:errorcluster, "AI2 Y Sum Set 1"=w992:i16, "AI2 Y Sum Set 2"=w991:i16, "AI1 X Set 1"=w763:fxp<+/-,16,1>, "AI1 X Set 2"=w762:fxp<+/-,16,1>, "Trap Pos FB Int Signal"=→"Trap Pos FB Int Signal":fxp<+/-,24,9>, "Trap Pos FB Int-Norm Signal"=→"Trap Pos FB Int-Norm Signal":fxp<+/-,16,1>, "Trap Pos FB Action"=w756:i64, "Scanning"=→"AOD Scanning":bool, "Scan I"=→"AOD Scan I":u64, "Scanning MCL"=w994:bool, "Scan I (MCL)"=→"MCL Scan I":u64, "Green FB Signals"=w931:T32)  [unwired: 1 out]
    "MCL Scanning" <- w994
    "Trap Pos FB Action" <- w756
    n706 = local read "AI2 (V)"() -> (w993:cluster{"Set 1":dbl, "Set 2":dbl})
    n707 = Bundle By Name(cluster=w993, "Set 1"=w992, "Set 2"=w991) -> (w989:cluster{"Set 1":dbl, "Set 2":dbl})
    n708 = Divide(x=w756, y=327.67) -> (x/y=→"Action (%)":dbl)
    n709 = local read "Trap X (AI1)"() -> (w776:T10)
    n710 = Divide(x=w989, y=3276.7) -> (x/y=w988:cluster{"Set 1":dbl, "Set 2":dbl})
    n711 = local write "AI2 (V)"(w988) -> ()
    n712 = Bundle(cluster=w776, "Trap 1"=w763, "Trap 2"=w762) -> (→"Trap X (AI1)":T10)
    n713 = Divide(x=w931, y=3276.7) -> (x/y=w927:T41)
    n714 = Unbundle By Name(w927) -> ("Green FB Ch 0"=w930:dbl, "Green FB Ch 1"=w929:dbl, "Green FB Ch 2"=w928:dbl)
    n715 = Divide(x=w930, y=w928) -> (x/y=w926:dbl)
    n716 = Divide(x=w929, y=w928) -> (x/y=w925:dbl)
    n717 = flat-sequence "To save data" {
      tunnel: [w3344] -> w1014
      tunnel: [w3345] -> w1013
      tunnel: w962 -> [w3338]
      tunnel: w847 -> [w3342]
      tunnel: ["Save Calibration"] -> w985
      tunnel: w982 -> [w3341]
      tunnel: [w3334] -> w981
      tunnel: [w3331] -> w980
      tunnel: [w3328] -> w979
      tunnel: w961 -> [w3330]
      tunnel: w866 -> [w3324]
      tunnel: [w3324] -> w865
      tunnel: ["Start Saving"] -> w821
      tunnel: [w3318] -> w744
      tunnel: [w3317] -> w743
      tunnel: w1014 -> [w3579]
      tunnel: w1013 -> [w3578]
      tunnel: w745 -> [w3577]
      tunnel: w985 -> [w3576]
      tunnel: w981 -> [w3574]
      tunnel: w980 -> [w3573]
      tunnel: w979 -> [w3572]
      tunnel: w834 -> [w3571]
      tunnel: w876 -> [w3570]
      tunnel: w865 -> [w3569]
      tunnel: w821 -> [w3568]
      tunnel: w819 -> [w3567]
      tunnel: w795 -> [w3566]
      tunnel: w744 -> [w3565]
      tunnel: w743 -> [w3564]
      tunnel: w742 -> [w3563]
      frame #0 {
        n718 = Or(x="Save N Sets", y="Start Saving") -> (x .or. y?=w3325:bool)
        n719 = To Double Precision Float(number=w3341) -> (double precision float=w3335:dbl)
        n720 = Build Array(w3325, "Save Calibration", w3338, w3330) -> (w3340:bool[])
        n721 = Compound Arithmetic op=OR("Save Calibration", w3338, w3325, w3330) -> (w3343:bool)
        n722 = Boolean Array To Number(Boolean array=w3340) -> (number=w3337:u32)
        n723 = feedback #19(FALSE ("Save APD Data\nwith Trap Data")) -> (w3319:bool)
        n724 = feedback #20(refnum<k0> refnum) -> (w3346:refnum<file>)
        n725 = feedback #21(refnum<k0> refnum) -> (w3321:refnum<file>)
        n726 = feedback #22(FALSE ("Save APD Data\nwith Trap Data")) -> (w3329:bool)
        n727 = feedback #23(refnum<k0> refnum) -> (w3332:refnum<file>)
        n728 = feedback #24(0) -> (w3348:i32)
        n729 = feedback #25() -> (w3336:u32)  [unwired: 1 out]
        n730 = case shown="True" w3343 {
          tunnel: [w3355 1] -> w3344
          tunnel: w3348 -> [w3357 _]
          tunnel: [w3356 w3375] -> w3345
          tunnel: w3346 -> [w3356 _]
          tunnel: w3342 -> [_ w3395]
          tunnel: w3335 -> [_ w3393]
          tunnel: w3337 -> [_ w3396]
          tunnel: [w3354 w3374] -> w3334
          tunnel: w3336 -> [w3354 _]
          tunnel: [w3353 w3372] -> w3331
          tunnel: w3332 -> [w3353 _]
          tunnel: [w3352 w3371] -> w3328
          tunnel: w3329 -> [w3352 _]
          tunnel: "Start Saving" -> [_ w3369]
          tunnel: w3324 -> [_ w3368]
          tunnel: [w3351 w3359] -> w3317
          tunnel: w3321 -> [w3351 _]
          tunnel: [w3350 w3358] -> w3318
          tunnel: w3319 -> [w3350 _]
          frame #0 {
            n731 = Increment(x=w3357) -> (x+1=w3355:i32)
          }
          frame #1 {
            w3365 = FALSE ("Start Saving")
            w3370 = 9.0  # File Version
            w3378 = FALSE ("prepend array or string size? (T)")
            w3376 = T34."big-endian, network order" ("byte order (0:big-endian, network order)")
            n732 = Array Size(array=w3368) -> (size(s)=w3367:i32)
            n733 = local read "BD 1 Frequency 1 (MHz)"() -> (w3392:dbl)
            n734 = local read "BD 2 Frequency 1 (MHz)"() -> (w3391:dbl)
            n735 = local read "BD 1 Frequency 2 (MHz)"() -> (w3390:dbl)
            n736 = local read "BD 2 Frequency 2 (MHz)"() -> (w3389:dbl)
            n737 = local read "BD 1 Frequency 3 (MHz)"() -> (w3388:dbl)
            n738 = local read "BD 2 Frequency 3 (MHz)"() -> (w3387:dbl)
            n739 = To Double Precision Float(number=w3367) -> (double precision float=w3366:dbl)
            n740 = local write "Save Calibration"(w3365) -> ()
            n741 = local write "Start Saving"(w3365) -> ()
            n742 = Build Array("Save APD Data\nwith Trap Data", "Save Trap Pos. Data") -> (w3362:bool[])
            n743 = Boolean Array To Number(Boolean array=w3362) -> (number=w3361:u32)
            n744 = Build Array(w3392, w3391, w3390, w3389, w3388, w3387) -> (w3386:dbl[])
            n745 = case shown="4" w3396 {
              tunnel: w3395 -> [w3467 w3487 w3503 w3541]
              tunnel: w3366 -> [w3472 w3494 w3523 w3560]
              tunnel: w3393 -> [w3471 w3493 w3522 w3559]
              tunnel: [w3468 w3489 w3514 w3551] -> w3384
              tunnel: [w3459 "Cal sets to save" w3504 w3542] -> w3374
              tunnel: w3386 -> [w3469 w3490 w3516 w3553]
              tunnel: "Save APD Data\nwith Trap Data" -> [w3466 _ w3500 w3539]
              tunnel: [w3466 w3481 w3500 w3539] -> w3371
              tunnel: w3370 -> [w3462 w3482 w3498 w3537]
              tunnel: w3369 -> [w3461 _ _ _]
              tunnel: [w3452 w3481 w3497 w3527] -> w3358
              tunnel: "Save Trap Pos. Data" -> [w3452 _ w3497 w3527]
              tunnel: w3361 -> [w3451 _ w3496 w3526]
              frame #0 {
                # "timeseries"
                n746 = case shown="True" "Profile" {
                  tunnel: [w3475 w3479] -> w3456
                  tunnel: [w3475 w3478] -> w3455
                  tunnel: [w3475 w3477] -> w3454
                  tunnel: [w3475 w3476] -> w3453
                  frame #0 {
                    w3475 = 0.0 ("f")
                  }
                  frame #1 {
                    n747 = local read "Current Position"() -> (w3480:cluster{dbl, dbl, dbl})
                    n748 = local read "Y change (mm)"() -> (w3476:dbl)
                    n749 = Unbundle(w3480) -> (w3479:dbl, w3478:dbl, w3477:dbl)
                  }
                }
                n750 = local read "Save ave N"() -> (w3474:dbl)
                n751 = Multiply(x=w3474, y=w3467) -> (x*y=w3473:dbl)
                n752 = To Double Precision Float(number=w3451) -> (double precision float=w3465:dbl)
                n753 = Build Array(w3462, w3467, w3473, w3472, w3471, 0.0 ("f")) -> (w3470:dbl[])
                n754 = Build Array(w3465, w3456, w3455, w3454, w3453) -> (w3463:dbl[])
                n755 = Select(t=u32 4000000000, s=w3461, f="N sets to save") -> (s? t:f=w3459:u32)